vi "FlexMag - 24-03-2023.vi"() -> ()   [LabVIEW 2018] (continued)
                        }
                      }
                      frame True {
                      }
                    }
                  }
                }
              }
              frame #39 {
                n11088 = local read "ch2-1 transfer"() -> (w16424:bool)
                n11089 = case shown="True" w16424 {
                  frame False {
                  }
                  frame True {
                    n11090 = local read "ABORT"() -> (w16425:bool)
                    n11091 = case shown="False" w16425 {
                      frame False {
                        n11092 = local write "trns 2-1 led 18"(TRUE ("trns 1-2 led 1")) -> ()
                        n11093 = Wait (ms)(milliseconds to wait=u32 100) -> ()  [unwired: 1 out]
                      }
                      frame True {
                      }
                    }
                  }
                }
              }
              frame #40 {
                n11094 = local read "ch2-1 transfer"() -> (w16428:bool)
                n11095 = case shown="True" w16428 {
                  frame False {
                  }
                  frame True {
                    n11096 = local read "ABORT"() -> (w16429:bool)
                    n11097 = case shown="False" w16429 {
                      frame False {
                        n11098 = while {
                          i -> [w16434]
                          stop <- w16435 stop-if-true
                          n11099 = Greater Or Equal?(x=w16434, y=100) -> (x >= y?=w16432:bool)
                          n11100 = case shown="True" w16432 {
                            frame False {
                            }
                            frame True {
                              n11101 = local write "Warning Message"("Transfer process canceled!\nCH1 Trns Bp Left coulnt't be closed" ("Warning Message")) -> ()
                              n11102 = local write "trns error"(TRUE ("TRNS error")) -> ()
                            }
                          }
                          n11103 = local read "CH1_Trns_BP_Left_DI"() -> (w16430:bool)
                          n11104 = case shown="True" w16430 {
                            tunnel: [TRUE ("CH1_Trns_BP_Left_DO") FALSE ("CH1_Trns_BP_Left_DO")] -> w16431
                            frame False {
                            }
                            frame True {
                              n11105 = Wait Until Next ms Multiple(millisecond multiple=u32 200) -> ()  [unwired: 1 out]
                              n11106 = local write "CH1_Trns_BP_Left_DO"(FALSE ("TRNS error")) -> ()
                            }
                          }
                          n11107 = local read "ch2-1 transfer"() -> (w16438:bool)
                          n11108 = local read "ABORT"() -> (w16437:bool)
                          n11109 = Not(x=w16438) -> (.not. x?=w16436:bool)
                          n11110 = Compound Arithmetic op=OR(w16431, w16437, w16436) -> (w16435:bool)
                        }
                      }
                      frame True {
                      }
                    }
                  }
                }
              }
              frame #41 {
                n11111 = local read "ch2-1 transfer"() -> (w16445:bool)
                n11112 = case shown="True" w16445 {
                  frame False {
                  }
                  frame True {
                    n11113 = local read "ABORT"() -> (w16446:bool)
                    n11114 = case shown="False" w16446 {
                      frame False {
                        n11115 = local write "trns 2-1 led 19"(TRUE ("trns 1-2 led 1")) -> ()
                        n11116 = Wait (ms)(milliseconds to wait=u32 100) -> ()  [unwired: 1 out]
                      }
                      frame True {
                      }
                    }
                  }
                }
              }
              frame #42 {
                n11117 = local read "ch2-1 transfer"() -> (w16449:bool)
                n11118 = case shown="True" w16449 {
                  frame False {
                  }
                  frame True {
                    n11119 = local read "ABORT"() -> (w16450:bool)
                    n11120 = case shown="False" w16450 {
                      frame False {
                        n11121 = while {
                          i -> [w16455]
                          stop <- w16456 stop-if-true
                          n11122 = Greater Or Equal?(x=w16455, y=100) -> (x >= y?=w16453:bool)
                          n11123 = case shown="True" w16453 {
                            frame False {
                            }
                            frame True {
                              n11124 = local write "Warning Message"("Transfer process canceled!\nCH2 Trns Bp Right coulnt't be closed" ("Warning Message")) -> ()
                              n11125 = local write "trns error"(TRUE ("TRNS error")) -> ()
                            }
                          }
                          n11126 = local read "CH2_Trns_BP_Right_DI"() -> (w16451:bool)
                          n11127 = case shown="True" w16451 {
                            tunnel: [TRUE ("CH1_Trns_BP_Left_DO") FALSE ("CH1_Trns_BP_Left_DO")] -> w16452
                            frame False {
                            }
                            frame True {
                              n11128 = local write "CH2_Trns_BP_Right_DO"(FALSE ("TRNS error")) -> ()
                              n11129 = Wait Until Next ms Multiple(millisecond multiple=u32 200) -> ()  [unwired: 1 out]
                            }
                          }
                          n11130 = local read "ch2-1 transfer"() -> (w16459:bool)
                          n11131 = local read "ABORT"() -> (w16458:bool)
                          n11132 = Not(x=w16459) -> (.not. x?=w16457:bool)
                          n11133 = Compound Arithmetic op=OR(w16452, w16458, w16457) -> (w16456:bool)
                        }
                      }
                      frame True {
                      }
                    }
                  }
                }
              }
              frame #43 {
                n11134 = local read "ch2-1 transfer"() -> (w16466:bool)
                n11135 = case shown="True" w16466 {
                  frame False {
                  }
                  frame True {
                    n11136 = local read "ABORT"() -> (w16467:bool)
                    n11137 = case shown="False" w16467 {
                      frame False {
                        n11138 = local write "trns 2-1 led 20"(TRUE ("trns 1-2 led 1")) -> ()
                        n11139 = Wait (ms)(milliseconds to wait=u32 100) -> ()  [unwired: 1 out]
                      }
                      frame True {
                      }
                    }
                  }
                }
              }
              frame #44 {
                n11140 = local read "ch2-1 transfer"() -> (w16470:bool)
                n11141 = case shown="True" w16470 {
                  frame False {
                  }
                  frame True {
                    n11142 = local read "ABORT"() -> (w16471:bool)
                    n11143 = case shown="False" w16471 {
                      frame False {
                        n11144 = stacked-sequence {
                          frame #0 {
                            n11145 = local read "ch2-1 transfer"() -> (w16472:bool)
                            n11146 = case shown="True" w16472 {
                              frame False {
                              }
                              frame True {
                                n11147 = local write "CH1_Trns_Gv_Open_DO"(FALSE ("trns clear")) -> ()
                              }
                            }
                          }
                          frame #1 {
                            n11148 = while {
                              i -> [w16478]
                              stop <- w16479 stop-if-true
                              n11149 = Greater Or Equal?(x=w16478, y=600) -> (x >= y?=w16476:bool)
                              n11150 = case shown="True" w16476 {
                                frame False {
                                }
                                frame True {
                                n11151 = local write "Warning Message"("Transfer process canceled!\nCH1-CH2 Trns GV couldn't be closed" ("Warning Message")) -> ()
                                n11152 = local write "trns error"(TRUE ("TRNS error")) -> ()
                                }
                              }
                              n11153 = local read "CH1_Trns_Gv_Close_DI"() -> (w16474:bool)
                              n11154 = case shown="False" w16474 {
                                tunnel: [FALSE ("CH1_Trns_BP_Left_DO") TRUE ("CH1_Trns_BP_Left_DO")] -> w16475
                                frame False {
                                n11155 = local write "CH1_Trns_Gv_Close_DO"(TRUE ("TRNS error")) -> ()
                                n11156 = Wait Until Next ms Multiple(millisecond multiple=u32 200) -> ()  [unwired: 1 out]
                                }
                                frame True {
                                }
                              }
                              n11157 = local read "ch2-1 transfer"() -> (w16482:bool)
                              n11158 = local read "ABORT"() -> (w16481:bool)
                              n11159 = Not(x=w16482) -> (.not. x?=w16480:bool)
                              n11160 = Compound Arithmetic op=OR(w16475, w16481, w16480) -> (w16479:bool)
                            }
                          }
                        }
                      }
                      frame True {
                      }
                    }
                  }
                }
              }
              frame #45 {
                n11161 = local read "ch2-1 transfer"() -> (w16489:bool)
                n11162 = case shown="True" w16489 {
                  frame False {
                  }
                  frame True {
                    n11163 = local read "ABORT"() -> (w16490:bool)
                    n11164 = case shown="False" w16490 {
                      frame False {
                        n11165 = local write "trns 2-1 led 21"(TRUE ("trns 1-2 led 1")) -> ()
                        n11166 = Wait (ms)(milliseconds to wait=u32 100) -> ()  [unwired: 1 out]
                      }
                      frame True {
                      }
                    }
                  }
                }
              }
              frame #46 {
                n11167 = local read "ch2-1 transfer"() -> (w16493:bool)
                n11168 = case shown="True" w16493 {
                  frame False {
                  }
                  frame True {
                    n11169 = local read "ABORT"() -> (w16494:bool)
                    n11170 = case shown="False" w16494 {
                      frame False {
                        n11171 = local read "target chamber"() -> (w16495:dbl)
                        n11172 = Equal?(x=w16495, y=1.0) -> (x = y?=w16496:bool)
                        n11173 = case shown="True" w16496 {
                          frame False {
                          }
                          frame True {
                            n11174 = stacked-sequence {
                              frame #0 {
                                n11175 = local read "ch2-1 transfer"() -> (w16498:bool)
                                n11176 = case shown="True" w16498 {
                                frame False {
                                }
                                frame True {
                                n11177 = local write "CH1_PetCool_Up_DO"(FALSE ("trns clear")) -> ()
                                }
                                }
                              }
                              frame #1 {
                                n11178 = while {
                                i -> [w16504]
                                stop <- w16505 stop-if-true
                                n11179 = Greater Or Equal?(x=w16504, y=300) -> (x >= y?=w16502:bool)
                                n11180 = case shown="True" w16502 {
                                frame False {
                                }
                                frame True {
                                n11181 = local write "Warning Message"("Transfer process canceled!\nCH1 Petcool couldn't be down" ("Warning Message")) -> ()
                                n11182 = local write "trns error"(TRUE ("TRNS error")) -> ()
                                }
                                }
                                n11183 = local read "CH1_PetCool_Down_DI"() -> (w16500:bool)
                                n11184 = case shown="False" w16500 {
                                tunnel: [FALSE ("CH1_Trns_BP_Left_DO") TRUE ("CH1_Trns_BP_Left_DO")] -> w16501
                                frame False {
                                n11185 = local write "CH1_PetCool_Down_DO"(TRUE ("TRNS error")) -> ()
                                n11186 = Wait Until Next ms Multiple(millisecond multiple=u32 200) -> ()  [unwired: 1 out]
                                }
                                frame True {
                                }
                                }
                                n11187 = local read "ch2-1 transfer"() -> (w16508:bool)
                                n11188 = local read "ABORT"() -> (w16507:bool)
                                n11189 = Not(x=w16508) -> (.not. x?=w16506:bool)
                                n11190 = Compound Arithmetic op=OR(w16501, w16507, w16506) -> (w16505:bool)
                                }
                              }
                            }
                          }
                        }
                      }
                      frame True {
                      }
                    }
                  }
                }
              }
              frame #47 {
                n11191 = local read "ch2-1 transfer"() -> (w16515:bool)
                n11192 = case shown="True" w16515 {
                  frame False {
                  }
                  frame True {
                    n11193 = local read "ABORT"() -> (w16516:bool)
                    n11194 = case shown="False" w16516 {
                      frame False {
                        n11195 = local write "trns 2-1 led 22"(TRUE ("trns 1-2 led 1")) -> ()
                        n11196 = Wait (ms)(milliseconds to wait=u32 100) -> ()  [unwired: 1 out]
                      }
                      frame True {
                      }
                    }
                  }
                }
              }
              frame #48 {
                n11197 = local read "ch2-1 transfer"() -> (w16519:bool)
                n11198 = case shown="True" w16519 {
                  frame False {
                  }
                  frame True {
                    n11199 = local read "ABORT"() -> (w16520:bool)
                    n11200 = case shown="False" w16520 {
                      frame False {
                        n11201 = local read "target chamber"() -> (w16521:dbl)
                        n11202 = Equal?(x=w16521, y=1.0) -> (x = y?=w16522:bool)
                        n11203 = case shown="True" w16522 {
                          frame False {
                          }
                          frame True {
                            n11204 = stacked-sequence {
                              frame #0 {
                                n11205 = local read "ch2-1 transfer"() -> (w16524:bool)
                                n11206 = case shown="True" w16524 {
                                frame False {
                                }
                                frame True {
                                n11207 = local write "CH1_SRV1_Piston_Back_DO"(FALSE ("trns clear")) -> ()
                                }
                                }
                              }
                              frame #1 {
                                n11208 = while {
                                i -> [w16530]
                                stop <- w16531 stop-if-true
                                n11209 = Greater Or Equal?(x=w16530, y=200) -> (x >= y?=w16528:bool)
                                n11210 = case shown="True" w16528 {
                                frame False {
                                }
                                frame True {
                                n11211 = local write "Warning Message"("Transfer process canceled!\nCH1 Servo Piston couldn't be forward" ("Warning Message")) -> ()
                                n11212 = local write "trns error"(TRUE ("TRNS error")) -> ()
                                }
                                }
                                n11213 = local read "CH1_SRV1_Piston_For_DI"() -> (w16526:bool)
                                n11214 = case shown="False" w16526 {
                                tunnel: [FALSE ("CH1_Trns_BP_Left_DO") TRUE ("CH1_Trns_BP_Left_DO")] -> w16527
                                frame False {
                                n11215 = local write "CH1_SRV1_Piston_For_DO"(TRUE ("TRNS error")) -> ()
                                n11216 = Wait Until Next ms Multiple(millisecond multiple=u32 200) -> ()  [unwired: 1 out]
                                }
                                frame True {
                                }
                                }
                                n11217 = local read "ch2-1 transfer"() -> (w16534:bool)
                                n11218 = local read "ABORT"() -> (w16533:bool)
                                n11219 = Not(x=w16534) -> (.not. x?=w16532:bool)
                                n11220 = Compound Arithmetic op=OR(w16527, w16533, w16532) -> (w16531:bool)
                                }
                              }
                            }
                          }
                        }
                      }
                      frame True {
                      }
                    }
                  }
                }
              }
              frame #49 {
                n11221 = local read "ch2-1 transfer"() -> (w16541:bool)
                n11222 = case shown="True" w16541 {
                  frame False {
                  }
                  frame True {
                    n11223 = local read "ABORT"() -> (w16542:bool)
                    n11224 = case shown="False" w16542 {
                      frame False {
                        n11225 = local write "trns 2-1 led 23"(TRUE ("trns 1-2 led 1")) -> ()
                        n11226 = Wait (ms)(milliseconds to wait=u32 100) -> ()  [unwired: 1 out]
                      }
                      frame True {
                      }
                    }
                  }
                }
              }
              frame #50 {
                n11227 = local read "ch2-1 transfer"() -> (w16545:bool)
                n11228 = case shown="True" w16545 {
                  frame False {
                  }
                  frame True {
                    n11229 = local read "ABORT"() -> (w16546:bool)
                    n11230 = case shown="False" w16546 {
                      frame False {
                        n11231 = disable-structure shown="Enabled" {
                          frame Disabled {
                            n11232 = stacked-sequence {
                              frame #0 {
                                n11233 = while {
                                i -> [w16551]
                                stop <- w16552 stop-if-true
                                n11234 = Greater Or Equal?(x=w16551, y=100) -> (x >= y?=w16549:bool)
                                n11235 = case shown="True" w16549 {
                                frame False {
                                }
                                frame True {
                                n11236 = local write "Warning Message"("Transfer process canceled!\nRight Slow Sensor problem" ("Warning Message")) -> ()
                                n11237 = local write "trns error"(TRUE ("TRNS error")) -> ()
                                }
                                }
                                n11238 = local read "Cnt_Right_Slow DI"() -> (w16547:bool)
                                n11239 = case shown="True" w16547 {
                                tunnel: [TRUE ("CH1_Trns_BP_Left_DO") FALSE ("CH1_Trns_BP_Left_DO")] -> w16548
                                frame False {
                                }
                                frame True {
                                n11240 = Wait Until Next ms Multiple(millisecond multiple=u32 200) -> ()  [unwired: 1 out]
                                n11241 = local write "Cnt_Right_Slow DO"(FALSE ("TRNS error")) -> ()
                                }
                                }
                                n11242 = local read "ch2-1 transfer"() -> (w16555:bool)
                                n11243 = local read "ABORT"() -> (w16554:bool)
                                n11244 = Not(x=w16555) -> (.not. x?=w16553:bool)
                                n11245 = Compound Arithmetic op=OR(w16548, w16554, w16553) -> (w16552:bool)
                                }
                              }
                              frame #1 {
                                n11246 = while {
                                i -> [w16566]
                                stop <- w16567 stop-if-true
                                n11247 = Greater Or Equal?(x=w16566, y=100) -> (x >= y?=w16564:bool)
                                n11248 = case shown="True" w16564 {
                                frame False {
                                }
                                frame True {
                                n11249 = local write "Warning Message"("Transfer process canceled!\nRight Limit Sensor problem" ("Warning Message")) -> ()
                                n11250 = local write "trns error"(TRUE ("TRNS error")) -> ()
                                }
                                }
                                n11251 = local read "Cnt_Right_Limit DI"() -> (w16562:bool)
                                n11252 = case shown="True" w16562 {
                                tunnel: [TRUE ("CH1_Trns_BP_Left_DO") FALSE ("CH1_Trns_BP_Left_DO")] -> w16563
                                frame False {
                                }
                                frame True {
                                n11253 = Wait Until Next ms Multiple(millisecond multiple=u32 200) -> ()  [unwired: 1 out]
                                n11254 = local write "Cnt_Right_Limit DO"(FALSE ("TRNS error")) -> ()
                                }
                                }
                                n11255 = local read "ch2-1 transfer"() -> (w16570:bool)
                                n11256 = local read "ABORT"() -> (w16569:bool)
                                n11257 = Not(x=w16570) -> (.not. x?=w16568:bool)
                                n11258 = Compound Arithmetic op=OR(w16563, w16569, w16568) -> (w16567:bool)
                                }
                              }
                              frame #2 {
                                n11259 = while {
                                i -> [w16581]
                                stop <- w16582 stop-if-true
                                n11260 = Greater Or Equal?(x=w16581, y=100) -> (x >= y?=w16579:bool)
                                n11261 = case shown="True" w16579 {
                                frame False {
                                }
                                frame True {
                                n11262 = local write "Warning Message"("Transfer process canceled!\nLeft Slow Sensor problem" ("Warning Message")) -> ()
                                n11263 = local write "trns error"(TRUE ("TRNS error")) -> ()
                                }
                                }
                                n11264 = local read "Cnt_Left_Slow DI"() -> (w16577:bool)
                                n11265 = case shown="True" w16577 {
                                tunnel: [TRUE ("CH1_Trns_BP_Left_DO") FALSE ("CH1_Trns_BP_Left_DO")] -> w16578
                                frame False {
                                }
                                frame True {
                                n11266 = Wait Until Next ms Multiple(millisecond multiple=u32 200) -> ()  [unwired: 1 out]
                                n11267 = local write "Cnt_Left_Slow DO"(FALSE ("TRNS error")) -> ()
                                }
                                }
                                n11268 = local read "ch2-1 transfer"() -> (w16585:bool)
                                n11269 = local read "ABORT"() -> (w16584:bool)
                                n11270 = Not(x=w16585) -> (.not. x?=w16583:bool)
                                n11271 = Compound Arithmetic op=OR(w16578, w16584, w16583) -> (w16582:bool)
                                }
                              }
                              frame #3 {
                                n11272 = while {
                                i -> [w16596]
                                stop <- w16597 stop-if-true
                                n11273 = Greater Or Equal?(x=w16596, y=100) -> (x >= y?=w16594:bool)
                                n11274 = case shown="True" w16594 {
                                frame False {
                                }
                                frame True {
                                n11275 = local write "Warning Message"("Transfer process canceled!\nLeft Limit Sensor problem" ("Warning Message")) -> ()
                                n11276 = local write "trns error"(TRUE ("TRNS error")) -> ()
                                }
                                }
                                n11277 = local read "Cnt_Left_Limit DI"() -> (w16592:bool)
                                n11278 = case shown="True" w16592 {
                                tunnel: [TRUE ("CH1_Trns_BP_Left_DO") FALSE ("CH1_Trns_BP_Left_DO")] -> w16593
                                frame False {
                                }
                                frame True {
                                n11279 = Wait Until Next ms Multiple(millisecond multiple=u32 200) -> ()  [unwired: 1 out]
                                n11280 = local write "Cnt_Left_Limit DO"(FALSE ("TRNS error")) -> ()
                                }
                                }
                                n11281 = local read "ch2-1 transfer"() -> (w16600:bool)
                                n11282 = local read "ABORT"() -> (w16599:bool)
                                n11283 = Not(x=w16600) -> (.not. x?=w16598:bool)
                                n11284 = Compound Arithmetic op=OR(w16593, w16599, w16598) -> (w16597:bool)
                                }
                              }
                            }
                          }
                          frame Enabled {
                            w16608 = FALSE ("CH4_SRV1_Piston_For_DO")
                            w16609 = FALSE ("CH4_SRV1_Piston_For_DO")
                            n11285 = local write "CH1_Right_Limit_DO"(w16609) -> ()
                            n11286 = local write "CH1_Right_Slow_DO"(w16609) -> ()
                            n11287 = local write "CH2_Right_Limit_DO"(w16609) -> ()
                            n11288 = local write "CH2_Right_Slow_DO"(w16609) -> ()
                            n11289 = local write "CH2_Left_Slow_DO"(w16609) -> ()
                            n11290 = local write "CH2_Left_Limit_DO"(w16609) -> ()
                            n11291 = Wait (ms)(milliseconds to wait=u32 2000) -> ()  [unwired: 1 out]
                            n11292 = local write "CH3_Right_Limit_DO"(w16608) -> ()
                            n11293 = local write "CH3_Right_Slow_DO"(w16608) -> ()
                            n11294 = local write "CH3_Left_Slow_DO"(w16608) -> ()
                            n11295 = local write "CH3_Left_Limit_DO"(w16608) -> ()
                            n11296 = local write "CH4_Left_Limit_DO"(w16608) -> ()
                            n11297 = local write "CH4_Left_Slow_DO"(w16608) -> ()
                          }
                        }
                      }
                      frame True {
                      }
                    }
                  }
                }
              }
              frame #51 {
                n11298 = local read "ch2-1 transfer"() -> (w16610:bool)
                n11299 = case shown="True" w16610 {
                  frame False {
                  }
                  frame True {
                    n11300 = local read "ABORT"() -> (w16611:bool)
                    n11301 = case shown="False" w16611 {
                      frame False {
                        n11302 = local write "trns 2-1 led 24"(TRUE ("trns 1-2 led 17")) -> ()
                        n11303 = Wait (ms)(milliseconds to wait=u32 100) -> ()  [unwired: 1 out]
                      }
                      frame True {
                      }
                    }
                  }
                }
              }
              frame #52 {
                n11304 = local read "ch2-1 transfer"() -> (w16614:bool)
                n11305 = case shown="True" w16614 {
                  frame False {
                  }
                  frame True {
                    n11306 = local read "ABORT"() -> (w16615:bool)
                    n11307 = case shown="False" w16615 {
                      frame False {
                        n11308 = local write "Buzzer DO"(TRUE ("trns 1-2 led 17")) -> ()
                        n11309 = Wait (ms)(milliseconds to wait=u32 3000) -> ()  [unwired: 1 out]
                        n11310 = local write "System Status"("CH2 to CH1  Transfer Completed" ("System Status")) -> ()
                      }
                      frame True {
                      }
                    }
                  }
                }
              }
              frame #53 {
                n11311 = local read "ch2-1 transfer"() -> (w16619:bool)
                n11312 = case shown="True" w16619 {
                  frame False {
                  }
                  frame True {
                    n11313 = local read "ABORT"() -> (w16620:bool)
                    n11314 = case shown="False" w16620 {
                      frame False {
                        w16621 = u16 1 items=["CH1"=1, "CH2"=2, "CH3"=3, "CH4"=4] ("cassette position selection")
                        w16622 = FALSE ("trns 1-2 led 17")
                        n11315 = Wait (ms)(milliseconds to wait=u32 1000) -> ()  [unwired: 1 out]
                        n11316 = local write "ch2-1 transfer"(FALSE ("trns 1-2 led 17")) -> ()
                        n11317 = local write "Buzzer DO"(FALSE ("trns 1-2 led 17")) -> ()
                        n11318 = local write "cassette position selection"(w16621) -> ()
                        n11319 = local write "System Status"("SEMI-AUTOMATIC MODE " ("System Status")) -> ()
                        n11320 = Not(x=w16622) -> (.not. x?=w16623:bool)
                        n11321 = local write "present location"(1.0 ("present location")) -> ()
                        n11322 = local write "casette_ch1_gui"(w16623) -> ()
                        n11323 = local write "casette_ch2_gui"(w16622) -> ()
                        n11324 = local write "casette_ch3_gui"(w16622) -> ()
                        n11325 = local write "casette_ch4_gui"(w16622) -> ()
                      }
                      frame True {
                      }
                    }
                  }
                }
              }
              frame #54 {
              }
            }
          }
          frame True {
          }
        }
      }
      frame 5 {
        n11326 = local read "ABORT"() -> (w16629:bool)
        n11327 = case shown="False" w16629 {
          frame False {
            n11328 = stacked-sequence {
              frame #0 {
                n11329 = local read "ch3-2 transfer"() -> (w16630:bool)
                n11330 = case shown="True" w16630 {
                  frame False {
                  }
                  frame True {
                    n11331 = local read "present location"() -> (w16633:dbl)
                    n11332 = Wait (ms)(milliseconds to wait=u32 100) -> ()  [unwired: 1 out]
                    n11333 = Equal?(x=w16633, y=3.0) -> (x = y?=w16634:bool)
                    n11334 = case shown="False" w16634 {
                      frame False {
                        n11335 = local write "trns error"(TRUE ("TRNS error")) -> ()
                        n11336 = local write "Warning Message"("Transfer process canceled!\nCassette is not in CH3" ("Warning Message")) -> ()
                      }
                      frame True {
                        n11337 = local write "System Status"("CH3 to CH2  Transfer in Progress" ("System Status")) -> ()
                      }
                    }
                  }
                }
              }
              frame #1 {
                n11338 = local read "ch3-2 transfer"() -> (w16638:bool)
                n11339 = case shown="True" w16638 {
                  frame False {
                  }
                  frame True {
                    n11340 = stacked-sequence {
                      frame #0 {
                        n11341 = local read "ABORT"() -> (w16639:bool)
                        n11342 = case shown="False" w16639 {
                          frame False {
                            n11343 = local write "trns pre check"(TRUE ("trns pre check")) -> ()
                          }
                          frame True {
                          }
                        }
                      }
                      frame #1 {
                        n11344 = Wait (ms)(milliseconds to wait=u32 1000) -> ()  [unwired: 1 out]
                      }
                      frame #2 {
                        n11345 = while {
                          i -> [w16647]
                          stop <- w16644 stop-if-true
                          # "10 min"
                          n11346 = local read "trns pre check"() -> (w16651:bool)
                          n11347 = local read "ch3-2 transfer"() -> (w16643:bool)
                          n11348 = local read "ABORT"() -> (w16645:bool)
                          n11349 = Greater Or Equal?(x=w16647, y=u32 2000 ("millisecond multiple")) -> (x >= y?=w16646:bool)
                          n11350 = Not(x=w16651) -> (.not. x?=w16650:bool)
                          n11351 = Not(x=w16643) -> (.not. x?=w16642:bool)
                          n11352 = Compound Arithmetic op=OR(w16646, w16650, w16645, w16642) -> (w16644:bool)
                          n11353 = Wait Until Next ms Multiple(millisecond multiple=u32 300) -> ()  [unwired: 1 out]
                        }
                      }
                    }
                  }
                }
              }
              frame #2 {
                n11354 = local read "ch3-2 transfer"() -> (w16652:bool)
                n11355 = case shown="True" w16652 {
                  frame False {
                  }
                  frame True {
                    n11356 = local read "trns V?"() -> (w16653:bool)
                    n11357 = case shown="False" w16653 {
                      frame False {
                        n11358 = stacked-sequence {
                          frame #0 {
                            n11359 = local read "ABORT"() -> (w16654:bool)
                            n11360 = case shown="False" w16654 {
                              frame False {
                                w16656 = FALSE ("CH1_CH_ATM_DO")
                                n11361 = local write "CH2_CH_ATM_DO"(w16656) -> ()
                                n11362 = local write "CH3_CH_ATM_DO"(w16656) -> ()
                                n11363 = Wait (ms)(milliseconds to wait=u32 3000) -> ()  [unwired: 1 out]
                              }
                              frame True {
                              }
                            }
                          }
                          frame #1 {
                            n11364 = while {
                              i -> [w16659]
                              stop <- w16660 stop-if-true
                              n11365 = Greater Or Equal?(x=w16659, y=200) -> (x >= y?=w16657:bool)
                              n11366 = case shown="True" w16657 {
                                frame False {
                                }
                                frame True {
                                n11367 = local write "Warning Message"("Transfer process canceled!\nChambers should be on Atmosphere Pressure" ("Warning Message")) -> ()
                                n11368 = local write "trns error"(TRUE ("TRNS error")) -> ()
                                }
                              }
                              n11369 = local read "CH2_CH_ATM_DI"() -> (w16664:bool)
                              n11370 = local read "CH3_CH_ATM_DI"() -> (w16663:bool)
                              n11371 = local read "ch3-2 transfer"() -> (w16666:bool)
                              n11372 = local read "ABORT"() -> (w16667:bool)
                              n11373 = Not(x=w16666) -> (.not. x?=w16665:bool)
                              n11374 = And(x=w16664, y=w16663) -> (x .and. y?=w16662:bool)
                              n11375 = Compound Arithmetic op=OR(w16662, w16667, w16665) -> (w16660:bool)
                              n11376 = Wait Until Next ms Multiple(millisecond multiple=u32 300) -> ()  [unwired: 1 out]
                            }
                          }
                        }
                      }
                      frame True {
                        n11377 = local read "ch2 ch pg torr"() -> (w16676:dbl)
                        n11378 = local read "ch3 ch pg torr"() -> (w16673:dbl)
                        n11379 = Greater Or Equal?(x=w16676, y=0.5) -> (x >= y?=w16672:bool)
                        n11380 = Greater Or Equal?(x=w16673, y=0.5) -> (x >= y?=w16671:bool)
                        n11381 = Or(x=w16672, y=w16671) -> (x .or. y?=w16670:bool)
                        n11382 = local write "trns error"(w16670) -> ()
                      }
                    }
                  }
                }
              }
              frame #3 {
                n11383 = local read "ch3-2 transfer"() -> (w16677:bool)
                n11384 = case shown="True" w16677 {
                  frame False {
                  }
                  frame True {
                    n11385 = local read "ABORT"() -> (w16678:bool)
                    n11386 = case shown="False" w16678 {
                      frame False {
                        n11387 = while {
                          i -> [w16683]
                          stop <- w16684 stop-if-true
                          n11388 = Greater Or Equal?(x=w16683, y=100) -> (x >= y?=w16681:bool)
                          n11389 = case shown="True" w16681 {
                            frame False {
                            }
                            frame True {
                              n11390 = local write "trns error"(TRUE ("TRNS error")) -> ()
                              n11391 = local write "Warning Message"("Transfer process canceled!\nCH2 Trns BP Left couln't be opened" ("Warning Message")) -> ()
                            }
                          }
                          n11392 = local read "CH2_Trns_BP_Left_DI"() -> (w16680:bool)
                          n11393 = case shown="False" w16680 {
                            tunnel: [FALSE ("CH1_Trns_BP_Left_DO") TRUE ("CH1_Trns_BP_Left_DO")] -> w16679
                            frame False {
                              n11394 = Wait Until Next ms Multiple(millisecond multiple=u32 200) -> ()  [unwired: 1 out]
                              n11395 = local write "CH2_Trns_BP_Left_DO"(TRUE ("CH1_Trns_BP_Left_DO")) -> ()
                            }
                            frame True {
                            }
                          }
                          n11396 = local read "ch3-2 transfer"() -> (w16687:bool)
                          n11397 = local read "ABORT"() -> (w16686:bool)
                          n11398 = Not(x=w16687) -> (.not. x?=w16685:bool)
                          n11399 = Compound Arithmetic op=OR(w16679, w16686, w16685) -> (w16684:bool)
                        }
                      }
                      frame True {
                      }
                    }
                  }
                }
              }
              frame #4 {
                n11400 = local read "ch3-2 transfer"() -> (w16694:bool)
                n11401 = case shown="True" w16694 {
                  frame False {
                  }
                  frame True {
                    n11402 = local read "ABORT"() -> (w16695:bool)
                    n11403 = case shown="False" w16695 {
                      frame False {
                        n11404 = local write "trns 3-2 led 1"(TRUE ("trns 1-2 led 1")) -> ()
                        n11405 = Wait (ms)(milliseconds to wait=u32 100) -> ()  [unwired: 1 out]
                      }
                      frame True {
                      }
                    }
                  }
                }
              }
              frame #5 {
                n11406 = local read "ch3-2 transfer"() -> (w16698:bool)
                n11407 = case shown="True" w16698 {
                  frame False {
                  }
                  frame True {
                    n11408 = local read "ABORT"() -> (w16699:bool)
                    n11409 = case shown="False" w16699 {
                      frame False {
                        n11410 = while {
                          i -> [w16704]
                          stop <- w16705 stop-if-true
                          n11411 = Greater Or Equal?(x=w16704, y=100) -> (x >= y?=w16702:bool)
                          n11412 = case shown="True" w16702 {
                            frame False {
                            }
                            frame True {
                              n11413 = local write "trns error"(TRUE ("TRNS error")) -> ()
                              n11414 = local write "Warning Message"("Transfer process canceled!\nCH3 Trns BP Right couln't be opened" ("Warning Message")) -> ()
                            }
                          }
                          n11415 = local read "CH3_Trns_BP_Right_DI"() -> (w16701:bool)
                          n11416 = case shown="False" w16701 {
                            tunnel: [FALSE ("CH1_Trns_BP_Left_DO") TRUE ("CH1_Trns_BP_Left_DO")] -> w16700
                            frame False {
                              n11417 = Wait Until Next ms Multiple(millisecond multiple=u32 200) -> ()  [unwired: 1 out]
                              n11418 = local write "CH3_Trns_BP_Right_DO"(TRUE ("CH1_Trns_BP_Left_DO")) -> ()
                            }
                            frame True {
                            }
                          }
                          n11419 = local read "ch3-2 transfer"() -> (w16708:bool)
                          n11420 = local read "ABORT"() -> (w16707:bool)
                          n11421 = Not(x=w16708) -> (.not. x?=w16706:bool)
                          n11422 = Compound Arithmetic op=OR(w16700, w16707, w16706) -> (w16705:bool)
                        }
                      }
                      frame True {
                      }
                    }
                  }
                }
              }
              frame #6 {
                n11423 = local read "ch3-2 transfer"() -> (w16715:bool)
                n11424 = case shown="True" w16715 {
                  frame False {
                  }
                  frame True {
                    n11425 = local read "ABORT"() -> (w16716:bool)
                    n11426 = case shown="False" w16716 {
                      frame False {
                        n11427 = local write "trns 3-2 led 2"(TRUE ("trns 1-2 led 1")) -> ()
                        n11428 = Wait (ms)(milliseconds to wait=u32 100) -> ()  [unwired: 1 out]
                      }
                      frame True {
                      }
                    }
                  }
                }
              }
              frame #7 {
                n11429 = local read "ch3-2 transfer"() -> (w16719:bool)
                n11430 = case shown="True" w16719 {
                  frame False {
                  }
                  frame True {
                    n11431 = local read "ABORT"() -> (w16720:bool)
                    n11432 = case shown="False" w16720 {
                      frame False {
                        n11433 = stacked-sequence {
                          frame #0 {
                            n11434 = local write "CH2_Trns_GV_Close_DO"(FALSE ("CH1_Trns_Gv_Close_DO")) -> ()
                            n11435 = Wait (ms)(milliseconds to wait=u32 100) -> ()  [unwired: 1 out]
                          }
                          frame #1 {
                            n11436 = while {
                              i -> [w16727]
                              stop <- w16728 stop-if-true
                              n11437 = Greater Or Equal?(x=w16727, y=600) -> (x >= y?=w16725:bool)
                              n11438 = case shown="True" w16725 {
                                frame False {
                                }
                                frame True {
                                n11439 = local write "trns error"(TRUE ("TRNS error")) -> ()
                                n11440 = local write "Warning Message"("Transfer process canceled!\nCH2-CH3 Trns GV couldn't be opened" ("Warning Message")) -> ()
                                }
                              }
                              n11441 = local read "CH2_Trns_Gv_Open_DI"() -> (w16724:bool)
                              n11442 = case shown="False" w16724 {
                                tunnel: [FALSE ("CH1_Trns_BP_Left_DO") TRUE ("CH1_Trns_BP_Left_DO")] -> w16723
                                frame False {
                                n11443 = local write "CH2_Trns_GV_Open_DO"(TRUE ("CH1_Trns_BP_Left_DO")) -> ()
                                n11444 = Wait Until Next ms Multiple(millisecond multiple=u32 200) -> ()  [unwired: 1 out]
                                }
                                frame True {
                                }
                              }
                              n11445 = local read "ch3-2 transfer"() -> (w16731:bool)
                              n11446 = local read "ABORT"() -> (w16730:bool)
                              n11447 = Not(x=w16731) -> (.not. x?=w16729:bool)
                              n11448 = Compound Arithmetic op=OR(w16723, w16730, w16729) -> (w16728:bool)
                            }
                          }
                        }
                      }
                      frame True {
                      }
                    }
                  }
                }
              }
              frame #8 {
                n11449 = local read "ch3-2 transfer"() -> (w16738:bool)
                n11450 = case shown="True" w16738 {
                  frame False {
                  }
                  frame True {
                    n11451 = local read "ABORT"() -> (w16739:bool)
                    n11452 = case shown="False" w16739 {
                      frame False {
                        n11453 = local write "trns 3-2 led 3"(TRUE ("trns 1-2 led 1")) -> ()
                        n11454 = Wait (ms)(milliseconds to wait=u32 100) -> ()  [unwired: 1 out]
                      }
                      frame True {
                      }
                    }
                  }
                }
              }
              frame #9 {
                n11455 = local read "ch3-2 transfer"() -> (w16742:bool)
                n11456 = case shown="True" w16742 {
                  frame False {
                  }
                  frame True {
                    n11457 = local read "ABORT"() -> (w16743:bool)
                    n11458 = case shown="False" w16743 {
                      frame False {
                        n11459 = while {
                          i -> [w16748]
                          stop <- w16749 stop-if-true
                          n11460 = Greater Or Equal?(x=w16748, y=100) -> (x >= y?=w16746:bool)
                          n11461 = case shown="True" w16746 {
                            frame False {
                            }
                            frame True {
                              n11462 = local write "trns error"(TRUE ("TRNS error")) -> ()
                              n11463 = local write "Warning Message"("Transfer process canceled!\nCH2 TGV Control Problem" ("Warning Message")) -> ()
                            }
                          }
                          n11464 = local read "CH2_TGV_Control_DI"() -> (w16745:bool)
                          n11465 = case shown="True" w16745 {
                            tunnel: [TRUE ("CH1_Trns_BP_Left_DO") FALSE ("CH1_Trns_BP_Left_DO")] -> w16744
                            frame False {
                            }
                            frame True {
                              n11466 = Wait Until Next ms Multiple(millisecond multiple=u32 200) -> ()  [unwired: 1 out]
                              n11467 = local write "CH2_TGV_Control_DO"(FALSE ("CH1_Trns_BP_Left_DO")) -> ()
                            }
                          }
                          n11468 = local read "ch3-2 transfer"() -> (w16752:bool)
                          n11469 = local read "ABORT"() -> (w16751:bool)
                          n11470 = Not(x=w16752) -> (.not. x?=w16750:bool)
                          n11471 = Compound Arithmetic op=OR(w16744, w16751, w16750) -> (w16749:bool)
                        }
                      }
                      frame True {
                      }
                    }
                  }
                }
              }
              frame #10 {
                n11472 = local read "ch3-2 transfer"() -> (w16759:bool)
                n11473 = case shown="True" w16759 {
                  frame False {
                  }
                  frame True {
                    n11474 = local read "ABORT"() -> (w16760:bool)
                    n11475 = case shown="False" w16760 {
                      frame False {
                        n11476 = local write "trns 3-2 led 4"(TRUE ("trns 1-2 led 1")) -> ()
                        n11477 = Wait (ms)(milliseconds to wait=u32 100) -> ()  [unwired: 1 out]
                      }
                      frame True {
                      }
                    }
                  }
                }
              }
              frame #11 {
                n11478 = local read "ch3-2 transfer"() -> (w16763:bool)
                n11479 = case shown="True" w16763 {
                  frame False {
                  }
                  frame True {
                    n11480 = local read "ABORT"() -> (w16764:bool)
                    n11481 = case shown="False" w16764 {
                      frame False {
                        n11482 = while {
                          i -> [w16769]
                          stop <- w16770 stop-if-true
                          n11483 = local read "CH1_Trns_Interlock_DI"() -> (w16765:bool)
                          n11484 = Greater Or Equal?(x=w16769, y=100) -> (x >= y?=w16767:bool)
                          n11485 = case shown="True" w16767 {
                            frame False {
                            }
                            frame True {
                              n11486 = local write "Warning Message"("Transfer process canceled!\nCH1 Interlock problem" ("Warning Message")) -> ()
                              n11487 = local write "trns error"(TRUE ("TRNS error")) -> ()
                            }
                          }
                          n11488 = case shown="False" w16765 {
                            tunnel: [w16774 TRUE ("CH1_Trns_BP_Left_DO")] -> w16766
                            frame False {
                              n11489 = local read "CH1_TGV_Control_DI"() -> (w16775:bool)
                              n11490 = case shown="False" w16775 {
                                tunnel: [FALSE ("CH1_Trns_BP_Left_DO") TRUE ("CH1_Trns_BP_Left_DO")] -> w16774
                                frame False {
                                n11491 = Wait Until Next ms Multiple(millisecond multiple=u32 200) -> ()  [unwired: 1 out]
                                n11492 = local write "CH1_TGV_Control_DO"(TRUE ("CH1_Trns_BP_Left_DO")) -> ()
                                }
                                frame True {
                                }
                              }
                            }
                            frame True {
                            }
                          }
                          n11493 = local read "ch3-2 transfer"() -> (w16773:bool)
                          n11494 = local read "ABORT"() -> (w16772:bool)
                          n11495 = Not(x=w16773) -> (.not. x?=w16771:bool)
                          n11496 = Compound Arithmetic op=OR(w16766, w16772, w16771) -> (w16770:bool)
                        }
                      }
                      frame True {
                      }
                    }
                  }
                }
              }
              frame #12 {
                n11497 = local read "ch3-2 transfer"() -> (w16783:bool)
                n11498 = case shown="True" w16783 {
                  frame False {
                  }
                  frame True {
                    n11499 = local read "ABORT"() -> (w16784:bool)
                    n11500 = case shown="False" w16784 {
                      frame False {
                        w16785 = TRUE ("CH3_Right_Limit_DO")
                        n11501 = local write "trns 3-2 led 5"(TRUE ("trns 1-2 led 1")) -> ()
                        n11502 = Wait (ms)(milliseconds to wait=u32 100) -> ()  [unwired: 1 out]
                        n11503 = local write "CH3_Right_Limit_DO"(w16785) -> ()
                        n11504 = local write "CH3_Right_Slow_DO"(w16785) -> ()
                        n11505 = local write "CH3_Left_Slow_DO"(w16785) -> ()
                        n11506 = local write "CH3_Left_Limit_DO"(w16785) -> ()
                      }
                      frame True {
                      }
                    }
                  }
                }
              }
              frame #13 {
                n11507 = local read "ch3-2 transfer"() -> (w16788:bool)
                n11508 = case shown="True" w16788 {
                  frame False {
                  }
                  frame True {
                    n11509 = local read "ABORT"() -> (w16789:bool)
                    n11510 = case shown="False" w16789 {
                      frame False {
                        n11511 = while {
                          i -> [w16794]
                          stop <- w16795 stop-if-true
                          n11512 = local read "CH3_Trns_Interlock_DI"() -> (w16790:bool)
                          n11513 = Greater Or Equal?(x=w16794, y=100) -> (x >= y?=w16792:bool)
                          n11514 = case shown="True" w16792 {
                            frame False {
                            }
                            frame True {
                              n11515 = local write "Warning Message"("Transfer process canceled!\nCH3 Interlock problem" ("Warning Message")) -> ()
                              n11516 = local write "trns error"(TRUE ("TRNS error")) -> ()
                            }
                          }
                          n11517 = case shown="False" w16790 {
                            tunnel: [w16799 TRUE ("CH1_Trns_BP_Left_DO")] -> w16791
                            frame False {
                              n11518 = local read "CH3_TGV_Control_DI"() -> (w16800:bool)
                              n11519 = case shown="False" w16800 {
                                tunnel: [FALSE ("CH1_Trns_BP_Left_DO") TRUE ("CH1_Trns_BP_Left_DO")] -> w16799
                                frame False {
                                n11520 = Wait Until Next ms Multiple(millisecond multiple=u32 200) -> ()  [unwired: 1 out]